vi "UHR-Fleezers Control (host) - Avogadro v1.vi"() -> ()   [LabVIEW 2014] (continued)
        n1782 = disable-structure shown="Disabled" {
          disable-tunnel: w2728 -> [w2730 _]
          frame Disabled {
            w2729 = FALSE ("Stop Flow")
            n1783 = local write "Stop Flow"(w2729) -> ()
            n1784 = local write "Sample Channel\nFlow"(w2729) -> ()
            n1785 = Concatenate Strings("stop" ("string"), "\r") -> (w2732:string)
            n1786 = VISA Write(VISA resource name=w2730, write buffer=w2732) -> ()  [unwired: 1 in, 3 out]
          }
          frame Enabled {
          }
        }
      }
      event "Flow rate (uL/h)": Value Change {
        n1787 = event-data() -> ()  [unwired: 7 out]
        n1788 = disable-structure shown="Disabled" {
          disable-tunnel: w2734 -> [w2736 _]
          frame Disabled {
            n1789 = Number To Decimal String(number="Flow rate (uL/h)") -> (decimal integer string=w2740:string)  [unwired: 1 in]
            n1790 = Concatenate Strings("irate  " ("string"), w2740, " u/h" ("string"), "\r") -> (w2739:string)
            n1791 = VISA Write(VISA resource name=w2736, write buffer=w2739) -> ()  [unwired: 1 in, 3 out]
          }
          frame Enabled {
          }
        }
      }
      event "Flush Sample": Value Change {
        n1792 = event-data() -> ()  [unwired: 7 out]
        n1793 = disable-structure shown="Disabled" {
          disable-tunnel: ["Flush Sample" _] -> w2743
          disable-tunnel: w2742 -> [w2749 _]
          frame Disabled {
            n1794 = flat-sequence {
              tunnel: w2749 -> [w2790]
              tunnel: [w2770] -> w2753
              tunnel: [w2766] -> w2752
              tunnel: ["Volume (uL)"] -> w2748
              tunnel: ["Flush rate (uL/m)"] -> w2747
              tunnel: w2753 -> [w2794]
              tunnel: [w2794] -> w2751
              tunnel: w2752 -> [w2793]
              tunnel: w2751 -> [w2799]
              frame #0 {
                # "set paramaters (rate, volume) for flush, clear volume"
                n1795 = Number To Decimal String(number="Flush rate (uL/m)") -> (decimal integer string=w2786:string)  [unwired: 1 in]
                n1796 = Concatenate Strings("irate  " ("string"), w2786, " u/m" ("string"), "\r") -> (w2788:string)
                n1797 = VISA Write(VISA resource name=w2790, write buffer=w2788) -> (VISA resource name out=w2784:refnum<visa-resource-name>)  [unwired: 1 in, 2 out]
                n1798 = Reciprocal(x="Flush rate (uL/m)") -> (1/x=w2769:dbl)
                n1799 = Number To Decimal String(number="Volume (uL)") -> (decimal integer string=w2775:string)  [unwired: 1 in]
                n1800 = Multiply(x="Volume (uL)", y=w2769) -> (x*y=w2768:dbl)
                n1801 = Concatenate Strings("tvolume  " ("string"), w2775, " u" ("string"), "\r") -> (w2773:string)
                n1802 = Multiply(x=w2768, y=60000.0) -> (x*y=w2766:dbl)
                n1803 = VISA Write(VISA resource name=w2784, write buffer=w2773) -> (VISA resource name out=w2772:refnum<visa-resource-name>)  [unwired: 1 in, 2 out]
                n1804 = Concatenate Strings("cvolume" ("string"), "\r") -> (w2771:string)
                n1805 = VISA Write(VISA resource name=w2772, write buffer=w2771) -> (VISA resource name out=w2782:refnum<visa-resource-name>)  [unwired: 1 in, 2 out]
                n1806 = Concatenate Strings("irun" ("string"), "\r") -> (w2780:string)
                n1807 = VISA Write(VISA resource name=w2782, write buffer=w2780) -> (VISA resource name out=w2770:refnum<visa-resource-name>)  [unwired: 1 in, 2 out]
              }
              frame #1 {
                # "Have to wait until\nflow is done to reset\nrate"
                n1808 = Add(x=w2793, y=100.0) -> (x+y=w2792:dbl)
                n1809 = Wait (ms)(milliseconds to wait=w2792) -> ()  [unwired: 1 out]
              }
              frame #2 {
                # "reset flow rate to usual flow rate"
                n1810 = local read "Flow rate (uL/h)"() -> (w2805:dbl)
                n1811 = Number To Decimal String(number=w2805) -> (decimal integer string=w2803:string)  [unwired: 1 in]
                n1812 = Concatenate Strings("irate  " ("string"), w2803, " u/h" ("string"), "\r") -> (w2801:string)
                n1813 = VISA Write(VISA resource name=w2799, write buffer=w2801) -> (VISA resource name out=w2795:refnum<visa-resource-name>)  [unwired: 1 in, 2 out]
                n1814 = Concatenate Strings("cvolume" ("string"), "\r") -> (w2796:string)
                n1815 = VISA Write(VISA resource name=w2795, write buffer=w2796) -> ()  [unwired: 1 in, 3 out]
              }
            }
            n1816 = local read "Save Event Log?"() -> (w2745:bool)
            n1817 = local read "Saving..."() -> (w2744:bool)
            n1818 = And(x=w2745, y=w2744) -> (x .and. y?=w2746:bool)
            n1819 = case shown="True" w2746 {
              tunnel: w2748 -> [_ w2755]
              tunnel: w2747 -> [_ w2754]
              frame False {
              }
              frame True {
                n1820 = Number To Decimal String(number=w2755) -> (decimal integer string=w2759:string)  [unwired: 1 in]
                n1821 = Number To Decimal String(number=w2754) -> (decimal integer string=w2761:string)  [unwired: 1 in]
                n1822 = local read "log file ref"() -> (w2756:refnum<file>)
                n1823 = local read "Time (s)"() -> (w2757:dbl)
                n1824 = Concatenate Strings("pump 2 flushing ", w2759, " uL at ", w2761, " ul/min") -> (w2763:string)
                n1825 = call "write to event log.vi"("log file ref"=w2756, "time"=w2757, "input string"=w2763) -> ()  [unwired: 8 in]
              }
            }
          }
          frame Enabled {
          }
        }
      }
      event "Flush Pump 3": Value Change {
        n1826 = event-data() -> ()  [unwired: 7 out]
        n1827 = disable-structure shown="Disabled" {
          disable-tunnel: ["Flush Pump 3" _] -> w2807
          disable-tunnel: w2806 -> [w2813 _]
          frame Disabled {
            n1828 = flat-sequence {
              tunnel: w2813 -> [w2828]
              tunnel: ["Flush rate (uL/m) P3"] -> w2809
              tunnel: ["Volume (uL) P3"] -> w2808
              frame #0 {
                # "set paramaters (rate, volume) for flush, clear volume"
                n1829 = Number To Decimal String(number="Flush rate (uL/m) P3") -> (decimal integer string=w2848:string)  [unwired: 1 in]
                n1830 = local write "Inject Pump 3"(TRUE ("Inject Pump 3")) -> ()
                n1831 = Concatenate Strings("irate  " ("string"), w2848, " u/m" ("string"), "\r") -> (w2850:string)
                n1832 = VISA Write(VISA resource name=w2828, write buffer=w2850) -> (VISA resource name out=w2846:refnum<visa-resource-name>)  [unwired: 1 in, 2 out]
                n1833 = Reciprocal(x="Flush rate (uL/m) P3") -> (1/x=w2832:dbl)
                n1834 = Number To Decimal String(number="Volume (uL) P3") -> (decimal integer string=w2837:string)  [unwired: 1 in]
                n1835 = Multiply(x="Volume (uL) P3", y=w2832) -> (x*y=w2831:dbl)
                n1836 = Concatenate Strings("tvolume  " ("string"), w2837, " u" ("string"), "\r") -> (w2835:string)
                n1837 = Multiply(x=w2831, y=60.0) -> (x*y=→"HP3 Flush Time (s)":dbl)
                n1838 = VISA Write(VISA resource name=w2846, write buffer=w2835) -> (VISA resource name out=w2834:refnum<visa-resource-name>)  [unwired: 1 in, 2 out]
                n1839 = Concatenate Strings("cvolume" ("string"), "\r") -> (w2833:string)
                n1840 = VISA Write(VISA resource name=w2834, write buffer=w2833) -> (VISA resource name out=w2844:refnum<visa-resource-name>)  [unwired: 1 in, 2 out]
                n1841 = Concatenate Strings("irun" ("string"), "\r") -> (w2842:string)
                n1842 = VISA Write(VISA resource name=w2844, write buffer=w2842) -> ()  [unwired: 1 in, 3 out]
              }
              frame #1 {
                "Flushing P3" <- TRUE ("Flushing P3")
              }
            }
            n1843 = local read "Save Event Log?"() -> (w2811:bool)
            n1844 = local read "Saving..."() -> (w2812:bool)
            n1845 = And(x=w2811, y=w2812) -> (x .and. y?=w2810:bool)
            n1846 = case shown="True" w2810 {
              tunnel: w2809 -> [_ w2816]
              tunnel: w2808 -> [_ w2815]
              frame False {
              }
              frame True {
                n1847 = Number To Decimal String(number=w2815) -> (decimal integer string=w2820:string)  [unwired: 1 in]
                n1848 = Number To Decimal String(number=w2816) -> (decimal integer string=w2822:string)  [unwired: 1 in]
                n1849 = local read "log file ref"() -> (w2817:refnum<file>)
                n1850 = local read "Time (s)"() -> (w2818:dbl)
                n1851 = Concatenate Strings("pump 3 flushing ", w2820, " uL at ", w2822, " ul/min") -> (w2824:string)
                n1852 = call "write to event log.vi"("log file ref"=w2817, "time"=w2818, "input string"=w2824) -> ()  [unwired: 8 in]
              }
            }
          }
          frame Enabled {
          }
        }
      }
      event "Flush Pump 1": Value Change {
        n1853 = event-data() -> ()  [unwired: 7 out]
        n1854 = disable-structure shown="Disabled" {
          disable-tunnel: ["Flush Pump 1" _] -> w2854
          disable-tunnel: w2853 -> [w2860 _]
          frame Disabled {
            n1855 = flat-sequence {
              tunnel: [w2881] -> w2862
              tunnel: w2860 -> [w2876]
              tunnel: ["Volume (uL) P1"] -> w2856
              tunnel: ["Flush rate (uL/m) P1"] -> w2855
              tunnel: w2862 -> [_]
              frame #0 {
                # "set paramaters (rate, volume) for flush, clear volume"
                n1856 = local write "Inject Pump 1"(TRUE ("Inject Pump 1")) -> ()
                n1857 = Number To Decimal String(number="Flush rate (uL/m) P1") -> (decimal integer string=w2897:string)  [unwired: 1 in]
                n1858 = Concatenate Strings("irate  " ("string"), w2897, " u/m" ("string"), "\r") -> (w2899:string)
                n1859 = VISA Write(VISA resource name=w2876, write buffer=w2899) -> (VISA resource name out=w2895:refnum<visa-resource-name>)  [unwired: 1 in, 2 out]
                n1860 = Reciprocal(x="Flush rate (uL/m) P1") -> (1/x=w2880:dbl)
                n1861 = Number To Decimal String(number="Volume (uL) P1") -> (decimal integer string=w2886:string)  [unwired: 1 in]
                n1862 = Multiply(x="Volume (uL) P1", y=w2880) -> (x*y=w2879:dbl)
                n1863 = Concatenate Strings("tvolume  " ("string"), w2886, " u" ("string"), "\r") -> (w2884:string)
                n1864 = Multiply(x=w2879, y=60.0) -> (x*y=→"HP1 Flush Time (s)":dbl)
                n1865 = VISA Write(VISA resource name=w2895, write buffer=w2884) -> (VISA resource name out=w2883:refnum<visa-resource-name>)  [unwired: 1 in, 2 out]
                n1866 = Concatenate Strings("cvolume" ("string"), "\r") -> (w2882:string)
                n1867 = VISA Write(VISA resource name=w2883, write buffer=w2882) -> (VISA resource name out=w2893:refnum<visa-resource-name>)  [unwired: 1 in, 2 out]
                n1868 = Concatenate Strings("irun" ("string"), "\r") -> (w2891:string)
                n1869 = VISA Write(VISA resource name=w2893, write buffer=w2891) -> (VISA resource name out=w2881:refnum<visa-resource-name>)  [unwired: 1 in, 2 out]
              }
              frame #1 {
                "Flushing P1" <- TRUE ("Flushing P3")
              }
            }
            n1870 = local read "Saving..."() -> (w2857:bool)
            n1871 = local read "Save Event Log?"() -> (w2858:bool)
            n1872 = And(x=w2858, y=w2857) -> (x .and. y?=w2859:bool)
            n1873 = case shown="True" w2859 {
              tunnel: w2856 -> [_ w2865]
              tunnel: w2855 -> [_ w2864]
              frame False {
              }
              frame True {
                n1874 = Number To Decimal String(number=w2865) -> (decimal integer string=w2869:string)  [unwired: 1 in]
                n1875 = Number To Decimal String(number=w2864) -> (decimal integer string=w2867:string)  [unwired: 1 in]
                n1876 = local read "log file ref"() -> (w2871:refnum<file>)
                n1877 = local read "Time (s)"() -> (w2872:dbl)
                n1878 = Concatenate Strings("pump 1 flushing ", w2869, " uL at ", w2867, " ul/min") -> (w2863:string)
                n1879 = call "write to event log.vi"("log file ref"=w2871, "time"=w2872, "input string"=w2863) -> ()  [unwired: 8 in]
              }
            }
          }
          frame Enabled {
          }
        }
      }
      event "Clear Volume": Value Change {
        n1880 = event-data() -> ()  [unwired: 7 out]
        n1881 = disable-structure shown="Disabled" {
          disable-tunnel: ["Clear Volume" _] -> w2903
          disable-tunnel: w2902 -> [w2904 _]
          frame Disabled {
            n1882 = Concatenate Strings("cvolume" ("string"), "\r") -> (w2905:string)
            n1883 = VISA Write(VISA resource name=w2904, write buffer=w2905) -> ()  [unwired: 1 in, 3 out]
          }
          frame Enabled {
          }
        }
      }
      event "Clear Volume P3": Value Change {
        n1884 = event-data() -> ()  [unwired: 7 out]
        n1885 = disable-structure shown="Disabled" {
          disable-tunnel: w2909 -> [w2911 _]
          frame Disabled {
            n1886 = Concatenate Strings("cvolume" ("string"), "\r") -> (w2912:string)
            n1887 = VISA Write(VISA resource name=w2911, write buffer=w2912) -> ()  [unwired: 1 in, 3 out]
            n1888 = local write "Clear Volume P3"(FALSE ("Clear Volume P3")) -> ()
          }
          frame Enabled {
          }
        }
      }
      event "Clear Volume P1": Value Change {
        n1889 = event-data() -> ()  [unwired: 7 out]
        n1890 = disable-structure shown="Disabled" {
          disable-tunnel: w2915 -> [w2917 _]
          frame Disabled {
            n1891 = Concatenate Strings("cvolume" ("string"), "\r") -> (w2918:string)
            n1892 = local write "Clear Volume P1"(FALSE ("Clear Volume P1")) -> ()
            n1893 = VISA Write(VISA resource name=w2917, write buffer=w2918) -> ()  [unwired: 1 in, 3 out]
          }
          frame Enabled {
          }
        }
      }
      event "Display On P3": Value Change {
        n1894 = event-data() -> ()  [unwired: 7 out]
        n1895 = disable-structure shown="Disabled" {
          disable-tunnel: w2921 -> [w2922 _]
          frame Disabled {
            n1896 = Select(t="dim 100", s="Display On P3", f="dim 0") -> (s? t:f=w2925:string)
            n1897 = Concatenate Strings(w2925, "\r") -> (w2927:string)
            n1898 = VISA Write(VISA resource name=w2922, write buffer=w2927) -> ()  [unwired: 1 in, 3 out]
          }
          frame Enabled {
          }
        }
      }
      event "Display On P1": Value Change {
        n1899 = event-data() -> ()  [unwired: 7 out]
        n1900 = disable-structure shown="Disabled" {
          disable-tunnel: w2929 -> [w2930 _]
          frame Disabled {
            n1901 = Select(t="dim 100", s="Display On P1", f="dim 0") -> (s? t:f=w2933:string)
            n1902 = Concatenate Strings(w2933, "\r") -> (w2935:string)
            n1903 = VISA Write(VISA resource name=w2930, write buffer=w2935) -> ()  [unwired: 1 in, 3 out]
          }
          frame Enabled {
          }
        }
      }
      event "Retract Pump 3": Value Change {
        n1904 = event-data() -> ()  [unwired: 7 out]
        n1905 = disable-structure shown="Disabled" {
          disable-tunnel: w2937 -> [w2938 _]
          frame Disabled {
            n1906 = local write "Retract Pump 3"(FALSE ("Retract Pump 3")) -> ()
            n1907 = case shown="True" "Retract Pump 3" {
              tunnel: w2938 -> [_ w2941]
              frame False {
              }
              frame True {
                n1908 = Number To Decimal String(number="Retract Rate (uL/m)") -> (decimal integer string=w2959:string)  [unwired: 1 in]
                n1909 = Concatenate Strings("wrate  " ("string"), w2959, " u/m" ("string"), "\r") -> (w2961:string)
                n1910 = VISA Write(VISA resource name=w2941, write buffer=w2961) -> (VISA resource name out=w2952:refnum<visa-resource-name>)  [unwired: 1 in, 2 out]
                n1911 = Number To Decimal String(number="Retract Vol 3 (uL)") -> (decimal integer string=w2954:string)  [unwired: 1 in]
                n1912 = Concatenate Strings("tvolume  " ("string"), w2954, " u" ("string"), "\r") -> (w2951:string)
                n1913 = VISA Write(VISA resource name=w2952, write buffer=w2951) -> (VISA resource name out=w2947:refnum<visa-resource-name>)  [unwired: 1 in, 2 out]
                n1914 = Concatenate Strings("cvolume" ("string"), "\r") -> (w2948:string)
                n1915 = VISA Write(VISA resource name=w2947, write buffer=w2948) -> (VISA resource name out=w2942:refnum<visa-resource-name>)  [unwired: 1 in, 2 out]
                n1916 = Concatenate Strings("wrun" ("string"), "\r") -> (w2943:string)
                n1917 = VISA Write(VISA resource name=w2942, write buffer=w2943) -> ()  [unwired: 1 in, 3 out]
              }
            }
          }
          frame Enabled {
          }
        }
      }
      event "Retract Pump 1": Value Change {
        n1918 = event-data() -> ()  [unwired: 7 out]
        n1919 = disable-structure shown="Disabled" {
          disable-tunnel: w2963 -> [w2964 _]
          frame Disabled {
            n1920 = local write "Retract Pump 1"(FALSE ("Retract Pump 1")) -> ()
            n1921 = case shown="True" "Retract Pump 1" {
              tunnel: w2964 -> [_ w2969]
              frame False {
              }
              frame True {
                n1922 = local read "Retract Rate (uL/m)"() -> (w2967:dbl)
                n1923 = Number To Decimal String(number=w2967) -> (decimal integer string=w2985:string)  [unwired: 1 in]
                n1924 = Concatenate Strings("wrate  " ("string"), w2985, " u/m" ("string"), "\r") -> (w2987:string)
                n1925 = VISA Write(VISA resource name=w2969, write buffer=w2987) -> (VISA resource name out=w2979:refnum<visa-resource-name>)  [unwired: 1 in, 2 out]
                n1926 = Number To Decimal String(number="Retract Vol 1 (uL)") -> (decimal integer string=w2981:string)  [unwired: 1 in]
                n1927 = Concatenate Strings("tvolume  " ("string"), w2981, " u" ("string"), "\r") -> (w2978:string)
                n1928 = VISA Write(VISA resource name=w2979, write buffer=w2978) -> (VISA resource name out=w2975:refnum<visa-resource-name>)  [unwired: 1 in, 2 out]
                n1929 = Concatenate Strings("cvolume" ("string"), "\r") -> (w2976:string)
                n1930 = VISA Write(VISA resource name=w2975, write buffer=w2976) -> (VISA resource name out=w2970:refnum<visa-resource-name>)  [unwired: 1 in, 2 out]
                n1931 = Concatenate Strings("wrun" ("string"), "\r") -> (w2971:string)
                n1932 = VISA Write(VISA resource name=w2970, write buffer=w2971) -> ()  [unwired: 1 in, 3 out]
              }
            }
          }
          frame Enabled {
          }
        }
      }
      event "Flip Green Filter": Value Change {
        n1933 = event-data() -> ()  [unwired: 7 out]
        n1934 = Not(x="Flip Green Filter") -> (.not. x?=w2990:bool)
        n1935 = local write "Flip Green Filter"(w2990) -> ()
        n1936 = flat-sequence {
          tunnel: [w2999] -> w2995
          tunnel: [w2998] -> w2994
          tunnel: w2989 -> [w2997]
          tunnel: [w3002] -> w2993
          tunnel: w2995 -> [w3002]
          tunnel: [w3001] -> w2992
          tunnel: w2994 -> [w3001]
          tunnel: w2993 -> [w3006]
          tunnel: w2992 -> [w3005]
          tunnel: [w3004] -> w2996
          frame #0 {
            n1937 = xnode "Read/Write Control"("FPGA VI Reference In"=w2997, "Green Filter Flipper"=TRUE) -> ("FPGA VI Reference Out"=w2999:T41, "error out"=w2998:errorcluster)  [unwired: 1 in]
          }
          frame #1 {
            n1938 = Wait (ms)(milliseconds to wait=u32 100) -> ()  [unwired: 1 out]
          }
          frame #2 {
            n1939 = xnode "Read/Write Control"("FPGA VI Reference In"=w3006, "error in"=w3005, "Green Filter Flipper"=FALSE) -> ("error out"=w3004:errorcluster)  [unwired: 1 out]
          }
        }
      }
      event "Pump 1 contents", "Pump 3 contents": Value Change {
        n1940 = event-data() -> ()  [unwired: 7 out]
        n1941 = local read "Pump 1 contents"() -> (→"Pump 1 cont disp":string)
        n1942 = local read "Pump 3 contents"() -> (→"Pump 3 cont disp":string)
      }
      event "Reset Trap Pos. FB": Value Change {
        n1943 = event-data() -> ()  [unwired: 7 out]
        n1944 = xnode "Read/Write Control"("FPGA VI Reference In"=w3010, "Trap Pos. FB Reset"="Reset Trap Pos. FB") -> ()  [unwired: 1 in, 2 out]
      }
      event "Rem fb disp offset": Value Change {
        n1945 = event-data() -> ()  [unwired: 7 out]
        n1946 = local write "Rem fb disp offset"(FALSE ("Rem fb disp offset")) -> ()
        n1947 = local read "Mean Trap Positions (nm)"() -> (w3013:T5)
        n1948 = local read "FB Trap Pos Offset"() -> (w3015:dbl)
        n1949 = Unbundle By Name(w3013) -> ("T1 X"=w3012:dbl)
        n1950 = Subtract(x=w3015, y=w3012) -> (x-y=w3014:dbl)
        n1951 = local write "FB Trap Pos Offset"(w3014) -> ()
      }
      event "Threshold (nm)": Value Change {
        n1952 = event-data() -> ()  [unwired: 7 out]
        n1953 = flat-sequence {
          tunnel: [w3020] -> w3018
          tunnel: w3017 -> [w3019]
          tunnel: w3018 -> [w3031]
          frame #0 {
            n1954 = xnode "Read/Write Control"("FPGA VI Reference In"=w3019) -> ("FPGA VI Reference Out"=w3023:T41, "error out"=w3022:errorcluster, "FPGA TTrig Thresh"=w3024:i64)  [unwired: 1 in]
            n1955 = local read "Threshold stored (nm)"() -> (w3030:dbl)
            n1956 = local read "Threshold (nm)"() -> (w3020:dbl)
            n1957 = local read "AOM X Cal (nm/MHz)"() -> (w3028:dbl)
            n1958 = Subtract(x=w3020, y=w3030) -> (x-y=w3029:dbl)
            n1959 = Divide(x=w3029, y=w3028) -> (x/y=w3026:dbl)
            n1960 = call "IR AOM freq to word.vi"("Frequency In (MHz)"=w3026) -> ("Frequency Word Out (double)"=w3027:dbl)
            n1961 = To Quad Integer(1:w3027) -> (0:w3025:i64)
            n1962 = Add(x=w3024, y=w3025) -> (x+y=w3021:i64)
            n1963 = xnode "Read/Write Control"("FPGA VI Reference In"=w3023, "error in"=w3022, "FPGA TTrig Thresh"=w3021) -> ()  [unwired: 2 out]
          }
          frame #1 {
            "Threshold stored (nm)" <- w3031
          }
        }
      }
      event "FB Trig Integrate": Value Change {
        n1964 = event-data() -> ()  [unwired: 7 out]
        n1965 = local read "FB Trig Integrate"() -> (w3034:u32)
        n1966 = xnode "Read/Write Control"("FPGA VI Reference In"=w3032, "FB Trig Integrate"=w3034) -> ("error out"=w3033:errorcluster)  [unwired: 1 in, 1 out]
      }
      event "11": Value Change {
        n1967 = event-data() -> ()  [unwired: 7 out]
        n1968 = local read "11"() -> (w3035:bool)
        n1969 = case shown="True" w3035 {
          frame False {
          }
          frame True {
            n1970 = local read "Messages"() -> (w3037:string)
            n1971 = call "Update messages.vi"("Message to add"="You kicked it up to 11!", "Old message string"=w3037) -> ("New message string"=w3038:string)
            n1972 = call <vilib>:"Beep.vi"() -> ()  [unwired: 12 in]
            n1973 = local write "Messages"(w3038) -> ()
          }
        }
      }
      event "Trap Pos. FB ON": Value Change {
        w3045 = 6.0  # clock mult.
        w3044 = 49152000.0  # TCXO frequ.
        n1974 = event-data() -> ()  [unwired: 7 out]
        n1975 = xnode "Read/Write Control"("FPGA VI Reference In"=w3039) -> ("FPGA VI Reference Out"=w3041:T41, "BD1 Frequency Out 1"=w3042:u64)  [unwired: 1 in, 1 out]
        n1976 = To Double Precision Float(number=w3042) -> (double precision float=w3046:dbl)
        n1977 = Multiply(x=w3044, y=w3045) -> (x*y=w3047:dbl)
        n1978 = Multiply(x=w3046, y=w3047) -> (x*y=w3048:dbl)
        n1979 = Scale By Power Of 2(n=-48, x=w3048) -> (x*2^n=w3050:dbl)
        n1980 = Divide(x=w3050, y=1000000.0) -> (x/y=w3043:dbl)
        n1981 = flat-sequence {
          tunnel: w3041 -> [w3056]
          tunnel: [w3055] -> w3052
          tunnel: "Trap Pos. FB ON" -> [w3054]
          tunnel: w3042 -> [w3053]
          tunnel: w3052 -> [w3062]
          tunnel: "Trap Pos. FB ON" -> [w3061]
          tunnel: w3043 -> [w3064]
          tunnel: "Trap Pos. FB ON" -> [w3063]
          frame #0 {
            n1982 = case shown="False" w3054 {
              tunnel: w3056 -> [w3058 w3060]
              tunnel: [w3059 w3060] -> w3055
              tunnel: w3053 -> [w3057 _]
              frame False {
                n1983 = xnode "Read/Write Control"("FPGA VI Reference In"=w3058, "BD 1 Frequency 1"=w3057) -> ("FPGA VI Reference Out"=w3059:T41)  [unwired: 1 in, 1 out]
              }
              frame True {
              }
            }
          }
          frame #1 {
            n1984 = xnode "Read/Write Control"("FPGA VI Reference In"=w3062, "Force feedback"=w3061) -> ()  [unwired: 1 in, 2 out]
          }
          frame #2 {
            n1985 = case shown="False" w3063 {
              tunnel: w3064 -> [w3065 _]
              frame False {
                n1986 = property on="BD 1 Frequency 1 (MHz)" class="DigNum (strict)"("Val(Sgnl)"=w3065) -> ()  [unwired: 2 in, 2 out]
              }
              frame True {
              }
            }
          }
        }
      }
      event "Remove Action Offset": Value Change {
        n1987 = event-data() -> ()  [unwired: 7 out]
        n1988 = local write "Remove Action Offset"(FALSE ("Remove Action Offset")) -> ()
        n1989 = local read "Trap Pos. FB Mult Factor"() -> (w3071:i64)
        n1990 = local read "Trap Pos FB Action"() -> (w3069:i64)
        n1991 = local read "Trap Pos. FB Offset Factor"() -> (w3067:i64)
        n1992 = Multiply(x=w3071, y=w3069) -> (x*y=w3070:i64)
        n1993 = Add(x=w3070, y=w3067) -> (x+y=w3068:i64)
        n1994 = local write "Trap Pos. FB Offset Factor"(w3068) -> ()
        n1995 = xnode "Read/Write Control"("FPGA VI Reference In"=w3066, "Trap Pos. FB Offset Factor"=w3068) -> ()  [unwired: 1 in, 2 out]
      }
      event "Remove Unwinding Offset": Value Change {
        n1996 = event-data() -> ()  [unwired: 7 out]
        n1997 = local write "Remove Unwinding Offset"(FALSE ("Remove Action Offset")) -> ()
        n1998 = local read "Trap Pos. FB Mult Factor"() -> (w3085:i64)
        n1999 = local read "Trap Pos FB Action"() -> (w3083:i64)
        n2000 = local read "Trap Pos. FB Offset Factor"() -> (w3082:i64)
        n2001 = Multiply(x=w3085, y=w3083) -> (x*y=w3084:i64)
        n2002 = local read "Trap Pos. FB Mult Factor"() -> (w3081:i64)
        n2003 = Add(x=w3084, y=w3082) -> (x+y=w3075:i64)
        n2004 = Multiply(x=32768, y="factor") -> (x*y=w3078:dbl)
        n2005 = Multiply(x=w3078, y=w3081) -> (x*y=w3080:dbl)
        n2006 = Subtract(x=w3075, y=w3080) -> (x-y=w3079:dbl)
        n2007 = To Quad Integer(1:w3079) -> (0:w3074:i64)
        n2008 = xnode "Read/Write Control"("FPGA VI Reference In"=w3073, "Trap Pos. FB Offset Factor"=w3074) -> ()  [unwired: 1 in, 2 out]
        n2009 = local write "Trap Pos. FB Offset Factor"(w3074) -> ()
      }
      event "Trap Pos. FB Range", "Trap Pos. FB Gains", "Trap Pos. FB Mult Factor", "Trap Pos. FB Offset Factor", "Trap Pos FB Negate Action", "Trap Pos FB Monitor\nT1 or T2", "Differential FB?", "Negate Diff?": Value Change {
        n2010 = event-data() -> ()  [unwired: 7 out]
        n2011 = local read "Negate Diff?"() -> (w3090:bool)
        n2012 = xnode "Read/Write Control"("FPGA VI Reference In"=w3089, "Trap Pos. FB Gains"="Trap Pos. FB Gains", "Trap pos. FB Range"="Trap Pos. FB Range", "Trap Pos. FB Mult Factor"="Trap Pos. FB Mult Factor", "Trap Pos. FB Offset Factor"="Trap Pos. FB Offset Factor", "Trap Pos FB Negate Action"="Trap Pos FB Negate Action", "Trap Pos FB Monitor T1 or T2"="Trap Pos FB Monitor\nT1 or T2", "AI1 X Scale"="Trap Pos. AI1 X Pre-scale", "Negate Diff?"=w3090, "Diff FB Measurement?"="Differential FB?") -> ()  [unwired: 1 in, 2 out]
      }
      event "Trap Pos FB SP", "Trap Pos FB SP 2", "Use SP 2": Value Change {
        n2013 = event-data() -> ()  [unwired: 7 out]
        n2014 = Select(t="Trap Pos FB SP 2", s="Use SP 2", f="Trap Pos FB SP") -> (s? t:f=w3098:fxp<+/-,16,1>)
        n2015 = xnode "Read/Write Control"("FPGA VI Reference In"=w3097, "Trap Pos. FB SP"=w3098) -> ()  [unwired: 1 in, 2 out]
      }
      event "Offset SP2 from SP1": Value Change {
        n2016 = event-data() -> ()  [unwired: 7 out]
        n2017 = local read "Trap Pos FB SP"() -> (w3104:fxp<+/-,16,1>)
        n2018 = Add(x=w3104, y="SP2 Offset") -> (x+y=w3102:fxp<+/-,16,1>)
        n2019 = property on="Trap Pos FB SP 2" class="DigNum (strict)"("Val(Sgnl)"=w3102) -> ()  [unwired: 2 in, 2 out]
        n2020 = local write "Offset SP2 from SP1"(FALSE ("Offset SP2 from SP1")) -> ()
      }
      event "Set Reading to\nSetpoint": Value Change {
        # "This is the actual PID input signal"
        n2021 = event-data() -> ()  [unwired: 7 out]
        n2022 = local write "Set Reading to\nSetpoint"(FALSE ("Set SP to Reading")) -> ()
        n2023 = xnode "Read/Write Control"("FPGA VI Reference In"=w3108) -> ("FPGA VI Reference Out"=w3111:T41, "error out"=w3110:errorcluster, "Trap Pos FB Int-Norm Signal"=w3109:fxp<+/-,16,1>, "BD1 Frequency Out 1"=w3107:u64)  [unwired: 1 in]
        n2024 = local read "Differential FB?"() -> (w3112:bool)
        n2025 = case shown="False" w3112 {
          tunnel: [w3141 w3148] -> w3106
          tunnel: w3109 -> [w3139 w3148]
          frame False {
            n2026 = local read "Trap Pos FB Monitor\nT1 or T2"() -> (w3144:bool)
            n2027 = local read "Trap X AI1 (DMA)"() -> (w3147:T19)
            n2028 = Unbundle By Name(w3147) -> ("Set 1"=w3146:fxp<+/-,16,1>, "Set 2"=w3145:fxp<+/-,16,1>)
            n2029 = Select(t=w3146, s=w3144, f=w3145) -> (s? t:f=w3143:fxp<+/-,16,1>)
            n2030 = Not(x="Set SP Using...") -> (.not. x?=w3140:bool)
            n2031 = Select(t=w3139, s=w3140, f=w3143) -> (s? t:f=w3141:fxp<+/-,16,1>)
          }
          frame True {
          }
        }
        n2032 = disable-structure shown="Disabled" {
          disable-tunnel: _ -> [w3117 _]
          disable-tunnel: w3107 -> [w3116 _]
          disable-tunnel: w3106 -> [w3115 _]
          frame Disabled {
            n2033 = case shown="True" w3117 {
              tunnel: [w3118 w3120] -> w3114
              tunnel: w3115 -> [w3118 w3119]
              tunnel: w3116 -> [_ w3138]
              frame False {
              }
              frame True {
                w3136 = 6.0  # clock mult.
                w3137 = 49152000.0  # TCXO frequ.
                # "Added by Ronen - for the real time\nchange of the setpoint to accomodate \nchanges in the offset."
                n2034 = To Double Precision Float(number=w3138) -> (double precision float=w3135:dbl)
                n2035 = local read "BD 1 Frequency 2 (MHz)"() -> (w3128:dbl)
                n2036 = Multiply(x=w3137, y=w3136) -> (x*y=w3134:dbl)
                n2037 = Multiply(x=w3135, y=w3134) -> (x*y=w3133:dbl)
                n2038 = local read "Offset file step size"() -> (w3126:dbl)
                n2039 = Scale By Power Of 2(n=-48, x=w3133) -> (x*2^n=w3131:dbl)
                n2040 = Divide(x=w3131, y=1000000.0) -> (x/y=w3129:dbl)
                n2041 = Subtract(x=w3128, y=w3129) -> (x-y=w3127:dbl)
                n2042 = Divide(x=w3127, y=w3126) -> (x/y=w3125:dbl)
                n2043 = local read item#-1() -> (w3123)
                n2044 = To Long Integer(number=w3125) -> (32bit integer=w3124:i32)
                n2045 = Index Array(array=w3123, index=w3124) -> (element=w3122)
                n2046 = To Fixed-Point(number=w3122) -> (fixed-point=w3121:fxp<+/-,16,1>)  [unwired: 1 in]
                n2047 = Add(x=w3119, y=w3121) -> (x+y=w3120:fxp<+/-,17,2>)
              }
            }
            "Offset corrected setpoint" <- w3114
          }
          frame Enabled {
          }
        }
        n2048 = local write "Trap Pos FB SP"(w3106) -> ()
        n2049 = xnode "Read/Write Control"("FPGA VI Reference In"=w3111, "error in"=w3110, "Trap Pos. FB SP"=w3106) -> ()  [unwired: 2 out]
      }
      event "Trap Pos. FB Out Scale 2^n": Value Change {
        n2050 = event-data() -> ()  [unwired: 7 out]
        n2051 = Scale By Power Of 2(n="Trap Pos. FB Out Scale 2^n", x=ext 1.0) -> (x*2^n=w3149:ext)
        n2052 = property on="Trap Pos. FB Mult Factor" class="DigNum (strict)"("Val(Sgnl)"=w3149) -> ()  [unwired: 2 in, 2 out]
      }
      event "Trap Pos FB Int Count": Value Change {
        n2053 = event-data() -> ()  [unwired: 7 out]
        n2054 = xnode "Read/Write Control"("FPGA VI Reference In"=w3152, "Trap Pos FB Int Count"="Trap Pos FB Int Count") -> ()  [unwired: 1 in, 2 out]
      }
      event "Display Saved Data": Value Change {
        n2055 = event-data() -> ()  [unwired: 7 out]
        n2056 = case shown="\"Amp Current\"" "Display Saved Data" {
          frame "Bead Seperation", Default {
            n2057 = property on="Amp current" class="WFGraph (strict)"("Visible"=FALSE) -> ()  [unwired: 2 in, 2 out]
            n2058 = property on="Trap Delta Graph" class="WFGraph (strict)"("Visible"=TRUE) -> ()  [unwired: 2 in, 2 out]
            n2059 = property on="Saved trap pos" class="WFGraph (strict)"("Visible"=FALSE) -> ()  [unwired: 2 in, 2 out]
          }
          frame "Amp Current" {
            n2060 = property on="Saved trap pos" class="WFGraph (strict)"("Visible"=FALSE) -> ()  [unwired: 2 in, 2 out]
            n2061 = property on="Trap Delta Graph" class="WFGraph (strict)"("Visible"=FALSE) -> ()  [unwired: 2 in, 2 out]
            n2062 = property on="Amp current" class="WFGraph (strict)"("Visible"=TRUE) -> ()  [unwired: 2 in, 2 out]
          }
          frame "Trap Position" {
            n2063 = property on="Saved trap pos" class="WFGraph (strict)"("Visible"=TRUE) -> ()  [unwired: 2 in, 2 out]
            n2064 = property on="Trap Delta Graph" class="WFGraph (strict)"("Visible"=FALSE) -> ()  [unwired: 2 in, 2 out]
            n2065 = property on="Amp current" class="WFGraph (strict)"("Visible"=FALSE) -> ()  [unwired: 2 in, 2 out]
          }
        }
      }
      event "Calibration": Value Change {
        n2066 = event-data() -> ()  [unwired: 7 out]
        n2067 = local read "X or Y?"() -> (w3180:bool)
        n2068 = local read "Calibration"() -> (w3177:u16)
        n2069 = Select(t="X" ("Label.Text"), s=w3180, f="Y" ("Label.Text")) -> (s? t:f=w3174:string)
        n2070 = case shown="0, Default" w3177 {
          tunnel: ["Position (V)" ("Label.Text") "Position (nm)" ("Label.Text") "Force (pN)" ("Label.Text")] -> w3171
          tunnel: [" (V)" ("Label.Text") " (nm)" ("Label.Text") " (pN)" ("Label.Text")] -> w3168
          frame 0, Default {
          }
          frame 1 {
          }
          frame 2 {
          }
        }
        n2071 = Concatenate Strings("T1 " ("Label.Text"), w3174) -> (w3170:string)
        n2072 = Concatenate Strings("T2 " ("Label.Text"), w3174) -> (w3169:string)
        n2073 = property on="Force" class="WFChart (strict)"("YScale.NameLbl.Text"=w3171) -> ()  [unwired: 2 in, 2 out]
        n2074 = Concatenate Strings("Mean" ("Label.Text"), w3168) -> (w3167:string)
        n2075 = Concatenate Strings(w3170, w3168) -> (w3166:string)
        n2076 = Concatenate Strings(w3169, w3168) -> (w3165:string)
        n2077 = Concatenate Strings("Difference" ("Label.Text"), w3168) -> (w3164:string)
        n2078 = property on="Mean" class="DigNum (strict)"("Caption.Text"=w3167) -> ()  [unwired: 2 in, 2 out]
        n2079 = property on="T1 X" class="DigNum (strict)"("Caption.Text"=w3166) -> ()  [unwired: 2 in, 2 out]
        n2080 = property on="T2 X" class="DigNum (strict)"("Caption.Text"=w3165) -> ()  [unwired: 2 in, 2 out]
        n2081 = property on="Difference" class="DigNum (strict)"("Caption.Text"=w3164) -> ()  [unwired: 2 in, 2 out]
      }
      event "Base N trap periods", "Period scale factor", "Trap osc amp (MHz)", "Cal sets to save", "# Samples/trap", "Total Counts (ticks)": Value Change {
        w3187 = 1.0
        w3193 = u32 0 ("y")
        # "scales 0 to 2pi"
        # "Create vector of trap offset (oscillation) values."
        # "Compute oscillation period as a multiple of the trap period. Should also fit nicely as a factor of the DMA period.\nCompare ticks for accurate commensurability check."
        # "Oscillation frequency needs to be commensurate\nwith the data save time."
        # "Be commensurate with total save time/100 (or so). That way you are guaranteed you can average spectra at least 100x."
        n2082 = event-data() -> ()  [unwired: 7 out]
        n2083 = local read "Total Counts (ticks)"() -> (w3209:u16)
        n2084 = To Unsigned Long Integer(number=w3209) -> (unsigned 32bit integer=w3219:u32)
        n2085 = Multiply "Base osc period (ticks)"(x=w3219, y="Base N trap periods") -> (x*y=w3210:u32)
        n2086 = local read "# Samples/trap"() -> (w3214:u32)
        n2087 = Multiply "Scaled osc period (ticks)"(x=w3210, y="Period scale factor") -> (x*y=w3211:dbl)
        n2088 = Multiply(x="Base N trap periods", y="Period scale factor") -> ()  [unwired: 1 out]
        n2089 = local read "Cal sets to save"() -> (w3215:u32)
        n2090 = To Unsigned Quad Integer(1:w3211) -> (0:w3201:u64)
        n2091 = for "vector 0 to N -1" {
          N: w3187 -> [_]
          tunnel: [w3236] -> w3207 mode=indexing
          i -> [w3236]
        }
        n2092 = Multiply "Ticks/DMA"(x=w3214, y=w3219) -> (x*y=w3218:u32)
        n2093 = Multiply "Scaled osc period (s)"(x=w3201, y=2.5e-08) -> (x*y=w3213:dbl)
        "Trap OSC Period (s)" <- w3213
        n2094 = Reciprocal(x=w3213) -> (1/x=→"A cal freq (Hz)":dbl)
        n2095 = Multiply(x=w3207, y=6.283185307179586) -> (x*y=w3222:dbl[])
        n2096 = Quotient & Remainder(x=w3218, y=w3201) -> (x-y*floor(x/y)=w3194:u64, floor(x/y)=→"N osc / DMA":u64)
        "DMA remainder" <- w3194
        n2097 = Multiply "Total trap ticks"(x=w3215, y=w3218) -> (x*y=w3202:u32)
        n2098 = Divide(x=w3222, y=w3187) -> (x/y=w3223:dbl[])
        n2099 = Sine(x=w3223) -> (sin(x)=w3224:dbl[])
        n2100 = Quotient & Remainder(x=w3202, y=100) -> (x-y*floor(x/y)=w3197:u32, floor(x/y)=w3217:u32)
        "Total save/100 remainder" <- w3197
        n2101 = Multiply "Single period osc vector"(x=w3224, y="Trap osc amp (MHz)") -> (x*y=w3200:dbl[])
        n2102 = Quotient & Remainder(x=w3217, y=w3201) -> (x-y*floor(x/y)=w3196:u64, floor(x/y)=→"N osc/ (total save/100)":u64)
        "(total save/100) /osc period remainder" <- w3196
        n2103 = Quotient & Remainder(x=w3202, y=w3201) -> (x-y*floor(x/y)=w3195:u64)  [unwired: 1 out]
        "N trap osc periods per save remainder" <- w3195
        n2104 = call "IR AOM freq to word - vec.vi"("Frequency In (double vec, MHz)"=w3200) -> ("Frequency Word Out"=w3199:dbl[])
        n2105 = To Quad Integer(1:w3199) -> (0:w3198:i64[])
        n2106 = disable-structure shown="Disabled" {
          disable-tunnel: w3206 -> [w3228 _]
          disable-tunnel: w3198 -> [w3226 _]
          frame Disabled {
            n2107 = xnode "Read/Write Control"("FPGA VI Reference In"=w3228) -> ("FPGA VI Reference Out"=w3227:T41)  [unwired: 3 in, 1 out]
            n2108 = flat-sequence {
              tunnel: w3226 -> [w3231]
              tunnel: w3227 -> [w3230]
              frame #0 {
                n2109 = for "Write data to fpga memory" {
                  tunnel: w3230 -> [w3233]
                  tunnel: w3231 -> [_] mode=indexing
                  (unwired) TRUE ("Ready Write")
                  n2110 = xnode "Read/Write Control"("FPGA VI Reference In"=w3233) -> ("FPGA VI Reference Out"=w3232:T41)  [unwired: 4 in, 1 out]
                  n2111 = while {
                    tunnel: w3232 -> [w3234]
                    stop <- _ continue-if-true
                    n2112 = xnode "Read/Write Control"("FPGA VI Reference In"=w3234) -> ()  [unwired: 1 in, 3 out]
                  }
                }
                "Writing waveform to fpga memory" <- TRUE ("Writing waveform to fpga memory")
              }
              frame #1 {
                n2113 = local write "Writing waveform to fpga memory"(FALSE ("Writing waveform to fpga memory")) -> ()
              }
            }
          }
          frame Enabled {
          }
        }
        n2114 = Equal?(x=w3196, y=w3193) -> (x = y?=w3191:bool)
        n2115 = Equal?(x=w3197, y=w3193) -> (x = y?=w3192:bool)
        n2116 = Equal?(x=w3194, y=w3193) -> (x = y?=w3189:bool)
        n2117 = Equal?(x=w3195, y=w3193) -> (x = y?=w3190:bool)
        n2118 = Compound Arithmetic op=AND(w3192, w3191, w3190, w3189) -> (→"Good freq?":bool)
      }
      event "Osc trap cont.", "Osc traps", "T1 Osc Enable", "T2 Osc Enable": Value Change {
        n2119 = event-data() -> ()  [unwired: 7 out]
        n2120 = disable-structure shown="Disabled" {
          disable-tunnel: w3237 -> [w3240 _]
          frame Disabled {
            n2121 = xnode "Read/Write Control"("FPGA VI Reference In"=w3240, "Trap 1 osc enable"="T1 Osc Enable", "Trap 2 osc enable"="T2 Osc Enable") -> ()  [unwired: 1 in, 2 out]
          }
          frame Enabled {
          }
        }
      }
      event "Pressure Pump Voltage (+/-10V)": Value Change {
        n2122 = event-data() -> ()  [unwired: 7 out]
        n2123 = disable-structure shown="Disabled" {
          disable-tunnel: w3241 -> [w3245 _]
          frame Disabled {
            n2124 = Divide(x="Pressure Pump Voltage (+/-10V)", y=10.0) -> (x/y=w3242:dbl)
            n2125 = Multiply(x=w3242, y=32767.0) -> (x*y=w3243:dbl)
            n2126 = xnode "Read/Write Control"("FPGA VI Reference In"=w3245, "Pressure Pump"=w3243) -> ()  [unwired: 1 in, 2 out]
          }
          frame Enabled {
          }
        }
      }
      event "Dynamic Force FB (ronen)": Value Change {
        # "Added by ronen - for feedback on trap position by changing the actual frequency and not the set frequency - for increasing the range of feedback."
        n2127 = event-data() -> ()  [unwired: 7 out]
        n2128 = xnode "Read/Write Control"("FPGA VI Reference In"=w3249, "Dynamic Force FB (Ronen)"="Dynamic Force FB (ronen)") -> ()  [unwired: 1 in, 2 out]
      }
      event "Read Setpoint Correction File": Value Change {
        n2129 = event-data() -> ()  [unwired: 7 out]
        n2130 = local write "Read Setpoint Correction File"(FALSE ("Read Setpoint Correction File")) -> ()
        n2131 = Open/Create/Replace File(file path (use dialog)="Setpoint Correction Offset File", operation (0:open)=T44."open", access (0:read/write)=enum16{"read/write", "read-only", "write-only"}."read-only") -> (refnum out=w3273:refnum<file>)  [unwired: 1 in, 4 out]
        n2132 = Deny Access(7:w3273) -> (3:w3272:refnum<file>)  [unwired: 1 in, 2 out]
        n2133 = Read from Binary File(5:0.0, 9:T45."big-endian, network order" ("byte order (0:big-endian, network order)"), 10:-1 ("count (1)"), 11:w3272) -> (2:w3266:dbl[], 3:w3271:refnum<file>)  [unwired: 1 in, 3 out]
        n2134 = Close File(refnum=w3271) -> ()  [unwired: 1 in, 2 out]
        n2135 = Array Subset(array=w3266, index=3) -> (w3267:dbl[])  [unwired: 1 in]
        n2136 = Index Array(array=w3266, index=0) -> (element=w3255:dbl)
        n2137 = local read "T2 calibration"() -> (w3250:T9)
        n2138 = local read "T1 calibration"() -> (w3262:T9)
        n2139 = local write "Offset file step size"(w3255) -> ()
        n2140 = Unbundle By Name(w3250) -> ("alpha_x (nm/V)"=w3257:dbl, "kappa_x (pN/nm)"=w3256:dbl)
        n2141 = Unbundle By Name(w3262) -> ("alpha_x (nm/V)"=w3259:dbl, "kappa_x (pN/nm)"=w3258:dbl)
        n2142 = Multiply(x=w3259, y=w3258) -> (x*y=w3260:dbl)
        n2143 = Multiply(x=w3257, y=w3256) -> (x*y=w3261:dbl)
        n2144 = Decimate 1D Array(w3267) -> (w3264:dbl[], w3263:dbl[])  [unwired: 1 out]
        n2145 = Divide(x=w3261, y=w3260) -> (x/y=w3252:dbl)
        n2146 = property on="B factor" class="DigNum (strict)"("Val(Sgnl)"=w3252) -> ()  [unwired: 2 in, 2 out]
        n2147 = Multiply(x=w3263, y=w3252) -> (x*y=w3265:dbl[])
        n2148 = Subtract(x=w3264, y=w3265) -> (x-y=w3251:dbl[])
        n2149 = local read "Offset Values"() -> (w3254:T20)
        n2150 = Bundle By Name(cluster=w3254, "Trap 1X offset"=w3264, "Trap 2X offset"=w3263) -> (w3253:T20)
        n2151 = local write "Offset Values"(w3253) -> ()
        n2152 = property on="Setpoint offset\ncorrection values" class="Arr (strict)"("Val(Sgnl)"=w3251) -> ()  [unwired: 2 in, 2 out]
      }
      event "B factor", "Setpoint offset\ncorrection values", "Target Force (pN)": Value Change {
        w3310 = 6.0  # clock mult.
        w3311 = 49152000.0  # TCXO frequ.
        n2153 = event-data() -> ()  [unwired: 7 out]
        n2154 = local read "B factor"() -> (w3312:dbl)
        n2155 = xnode "Read/Write Control"("FPGA VI Reference In"=w3313, "B factor"=w3312) -> ("BD1 Frequency Out 1"=w3303:u64)  [unwired: 1 in, 2 out]
        n2156 = To Double Precision Float(number=w3303) -> (double precision float=w3309:dbl)
        n2157 = local read "BD 1 Frequency 2 (MHz)"() -> (w3301:dbl)
        n2158 = Multiply(x=w3311, y=w3310) -> (x*y=w3308:dbl)
        n2159 = Multiply(x=w3309, y=w3308) -> (x*y=w3307:dbl)
        n2160 = Scale By Power Of 2(n=-48, x=w3307) -> (x*2^n=w3305:dbl)
        n2161 = Divide(x=w3305, y=1000000.0) -> (x/y=w3302:dbl)
        n2162 = Subtract(x=w3301, y=w3302) -> (x-y=w3289:dbl)
        n2163 = local read "Target Force (pN)"() -> (w3300:dbl)
        n2164 = local read "T1 calibration"() -> (w3298:T9)
        n2165 = local read "Offset file step size"() -> (w3288:dbl)
        n2166 = local read "Setpoint offset\ncorrection values"() -> (w3285:dbl[])
        n2167 = Unbundle By Name(w3298) -> ("alpha_x (nm/V)"=w3297:dbl, "kappa_x (pN/nm)"=w3296:dbl)
        n2168 = Multiply(x=w3300, y=2.0) -> (x*y=w3294:dbl)
        n2169 = Divide(x=w3289, y=w3288) -> (x/y=w3287:dbl)
        n2170 = local read "Negate Diff?"() -> (w3291:bool)
        n2171 = To Long Integer(number=w3287) -> (32bit integer=w3286:i32)
        n2172 = Multiply(x=w3297, y=w3296) -> (x*y=w3295:dbl)
        n2173 = Index Array(array=w3285, index=w3286) -> (element=w3283:dbl)
        n2174 = Divide(x=w3294, y=w3295) -> (x/y=w3290:dbl)
        n2175 = Select(t=1, s=w3291, f=-1) -> (s? t:f=w3284:i32)
        n2176 = Multiply(x=w3284, y=w3283) -> (x*y=w3282:dbl)
        n2177 = Add(x=w3290, y=w3282) -> (x+y=w3281:dbl)
        n2178 = To Fixed-Point(number=w3281) -> (fixed-point=w3280:fxp<+/-,16,1>)  [unwired: 1 in]
        n2179 = property on="Trap Pos FB SP" class="DigNum (strict)"("Val(Sgnl)"=w3280) -> ()  [unwired: 2 in, 2 out]
      }
      event "Trap 3 (ON/OFF)", "T3 Y (V)", "T3 X (V)": Value Change {
        n2180 = event-data() -> ()  [unwired: 7 out]
        n2181 = case shown="False" "Trap 3 (ON/OFF)" {
          tunnel: [5.0 0.0] -> w3315
          frame False {
          }
          frame True {
          }
        }
        n2182 = Multiply(x="T3 X (V)", y=32767.0) -> (x*y=w3331:dbl)
        n2183 = Multiply(x="T3 Y (V)", y=32767.0) -> (x*y=w3328:dbl)
        n2184 = Divide(x=w3331, y=10.0) -> (x/y=w3332:dbl)
        n2185 = Divide(x=w3328, y=10.0) -> (x/y=w3327:dbl)
        n2186 = To Word Integer(number=w3332) -> (16bit integer=w3321:i16)
        n2187 = To Word Integer(number=w3327) -> (16bit integer=w3322:i16)
        n2188 = Multiply(x=w3315, y=32767.0) -> (x*y=w3318:dbl)
        n2189 = Divide(x=w3318, y=10.0) -> (x/y=w3317:dbl)
        n2190 = To Word Integer(number=w3317) -> (16bit integer=w3314:i16)
        n2191 = xnode "Read/Write Control"("FPGA VI Reference In"=w3323, "Piezo Trap X (AO5)"=w3321, "Piezo Trap Y (AO4)"=w3322, "Piezo Trap ON/Off (AO3)"=w3314) -> ()  [unwired: 1 in, 2 out]
      }
      event "Cursor control.X", "Cursor control.Y": Value Change {
        # "If turning cursor control off, update the piezo controls"
        n2192 = event-data() -> ()  [unwired: 7 out]
        n2193 = xnode "Read/Write Control"("FPGA VI Reference In"=w3342) -> ("Piezo X out"=w3340:i16, "Piezo Y out"=w3336:i16)  [unwired: 1 in, 2 out]
        n2194 = local read "Cursor control"() -> (w3341:cluster{"X":bool, "Y":bool})
        n2195 = Unbundle By Name(w3341) -> ("X"=w3339:bool, "Y"=w3338:bool)
        n2196 = And(x=w3339, y=w3338) -> (x .and. y?=w3337:bool)
        n2197 = case shown="True" w3337 {
          tunnel: w3340 -> [w3347 _]
          tunnel: w3336 -> [w3345 _]
          frame False {
            w3344 = 3276.7
            n2198 = Divide(x=w3347, y=w3344) -> (x/y=w3346:dbl)
            n2199 = Divide(x=w3345, y=w3344) -> (x/y=w3343:dbl)
            n2200 = property on="T3 X (V)" class="DigNum (strict)"("Val(Sgnl)"=w3346) -> ()  [unwired: 2 in, 2 out]
            n2201 = property on="T3 Y (V)" class="DigNum (strict)"("Val(Sgnl)"=w3343) -> ()  [unwired: 2 in, 2 out]
          }
          frame True {
          }
        }
      }
    }
    "error out 2" <- w1706
    n2202 = node-c288() -> ()  [unwired: 2 out]
  }
  n2203 = node-c288() -> (w67:T35)  [unwired: 4 out]
  n2204 = timed-loop "Mouse control: trap position (AOM deflection), set confocal spot from image" {
    tunnel: [w3348] -> w72
    timing: w67 -> [_]
    timing-out: [_] -> w66
    tunnel: w25 -> [w3349]
    stop <- w3348 stop-if-true
    n2205 = node-c288() -> ()  [unwired: 2 out]
    n2206 = event shown="[0] \"Pane\": Mouse Down" {
      selector: _ -> [_ _ _ _]
      dyn-events: _ -> [_ _ _ _]
      timeout: _ -> [_ _ _ _]
      tunnel: w3349 -> [w3352 _ _ _]
      tunnel: [_ _ TRUE _] -> w3348
      event Mouse Down {
        n2207 = event-data() -> ("Time"=w3354:u32, "Coords"=w3353:T12, "Button"=w3355:u16)  [unwired: 6 out]
        n2208 = case shown="1" w3355 {
          tunnel: w3354 -> [_ _ w3480]
          tunnel: w3353 -> [_ w3392 w3478]
          tunnel: w3352 -> [_ _ w3474]
          frame 0, Default {
          }
          frame 1 {
            n2209 = property on="APD 2" class="ImageControl"() -> ("Displayed Image Position"=w3362:cluster{"Left":i32, "Top":i32})  [unwired: 2 in, 2 out]
            n2210 = property on="APD 1" class="ImageControl"() -> ("Displayed Image Position"=w3391:cluster{"Left":i32, "Top":i32})  [unwired: 2 in, 2 out]
            n2211 = property on="Detection Laser X" class="ImageControl"() -> ("Displayed Image Position"=w3388:cluster{"Left":i32, "Top":i32})  [unwired: 2 in, 2 out]
            n2212 = property on="Detection Laser Y" class="ImageControl"() -> ("Displayed Image Position"=w3387:cluster{"Left":i32, "Top":i32})  [unwired: 2 in, 2 out]
            n2213 = property on="APD 2" class="ImageControl"() -> ("Displayed Image Size"=w3361:cluster{"Width":u32, "Height":u32})  [unwired: 2 in, 2 out]
            n2214 = property on="APD 1" class="ImageControl"() -> ("Displayed Image Size"=w3389:cluster{"Width":u32, "Height":u32})  [unwired: 2 in, 2 out]
            n2215 = property on="Detection Laser X" class="ImageControl"() -> ("Displayed Image Size"=w3390:cluster{"Width":u32, "Height":u32})  [unwired: 2 in, 2 out]
            n2216 = property on="Detection Laser Y" class="ImageControl"() -> ("Displayed Image Size"=w3386:cluster{"Width":u32, "Height":u32})  [unwired: 2 in, 2 out]
            n2217 = Unbundle By Name(w3361) -> ("Width"=w3358:u32, "Height"=w3357:u32)
            n2218 = Unbundle By Name(w3362) -> ("Left"=w3360:i32, "Top"=w3359:i32)
            n2219 = Unbundle By Name(w3389) -> ("Width"=w3383:u32, "Height"=w3382:u32)
            n2220 = Unbundle By Name(w3390) -> ("Width"=w3379:u32, "Height"=w3378:u32)
            n2221 = Unbundle By Name(w3386) -> ("Width"=w3375:u32, "Height"=w3374:u32)
            n2222 = Unbundle By Name(w3391) -> ("Left"=w3385:i32, "Top"=w3384:i32)
            n2223 = Unbundle By Name(w3388) -> ("Left"=w3381:i32, "Top"=w3380:i32)
            n2224 = Unbundle By Name(w3387) -> ("Left"=w3377:i32, "Top"=w3376:i32)
            n2225 = Bundle("Left"=w3360, "Top"=w3359, "Width"=w3358, "Height"=w3357) -> (w3356:T50)  [unwired: 1 in]